vi "Configured Acquisition Trigger (Host)_20230131.vi"() -> ()   [LabVIEW 2021]
doc: "Use this VI as a template to design an application that acquires data using advanced triggering logic from the NI PXIe-5170R/5171R."
uses:
  <instrlib>/_niInstr/Multirecord Acquisition/Interface/v1/Host/Public/Full Record Status.ctl
  <instrlib>/_niInstr/Multirecord Acquisition/Interface/v1/Host/Public/Record State.ctl
  <instrlib>/_niInstr/Multirecord Acquisition/Interface/v1/Host/Public/Record Status.ctl
  Enums/Channel Numbers.ctl
  <instrlib>/_niInstr/Multirecord Acquisition/Interface/v1/Host/Public/Fetch Relative To Enum.ctl
  <vilib>/FPGAPlugInAG/PXIe-5172 (8CH - 410T)/niLvFpga_Open_PXIe-5172 (8CH - 410T).vi
  <vilib>/rvi/interface/common/dynamic/niFpgaDynamicAddResources.vi
  <vilib>/FPGAPlugInAG/Dynamic/niLvFpga_Close_Dynamic.vi
  <vilib>/rvi/interface/nirviOpenFPGA/nirviOpenFPGA.xnode
  FPGA Bitfiles/Multirecord Acquisition FPGA_20221228a_5.lvbitx
  <vilib>/rvi/interface/nirviCloseFPGA/nirviCloseFPGA.xnode
  Device Session/Device Session.lvclass
  <instrlib>/_niInstr/Multirecord Acquisition/Interface/v1/Host/niInstr Multirecord Acquisition v1 Host.lvclass
panel:
  in  "Increment Records":bool
  out "records done":u64[](array[numeric])
  out "current record status":T1
  out "fetch backlog":u64[](array[numeric])
  out "record status":T2
  out "done":bool
  out "Host Loop Count":i32
  out "Graph 1":T4(graph)
  out "TrigCfg Array":T5(array[cluster])
  out "TrigCount":u32[](array[numeric])
  in  "ResetTrig":bool=TRUE
  in  "Sliding Window Trigger":cluster{"Range":dbl, "StartCenter":dbl}[](array[cluster])=[{"Range"=0.2, "StartCenter"=0.0}, {"Range"=0.2, "StartCenter"=0.0}]
  out "actual sample rate":dbl format="%#_6p"
  in  "onboard sample clock rate":dbl(ring)=200000000.0 items=["250 MHz"=250000000.0, "200 MHz"=200000000.0, "150 MHz"=150000000.0]
  in  "impedance":enum8{"Default", "1 mega ohm", "50 ohm"}(ring)
  in  "vertical offset (V)":dbl format="%.2p"
  out "Graph 0":T4(graph)
  in  "mode":T6(ring)
  in  "decimation factor":u16=1
  in  "coupling":enum8{"Default", "DC", "AC"}(ring)
  in  "bandwidth":T7(ring)
  in  "pretrigger samples":u64=500
  in  "number of samples":u64=1000
  in  "RIO Device":tag="PXI1Slot8"
  in  "channel(s)":string="0,1"
  in  "vertical range (Vpp)":dbl=2.0 format="%.2p"
  out "error out":errorcluster
  in  "stop":bool
  # "RIO Device"
  # "Vertical Settings"
  # "Trigger Settings"
  # "Acquisition Settings"
  # "DSP"
  # "Clocking"
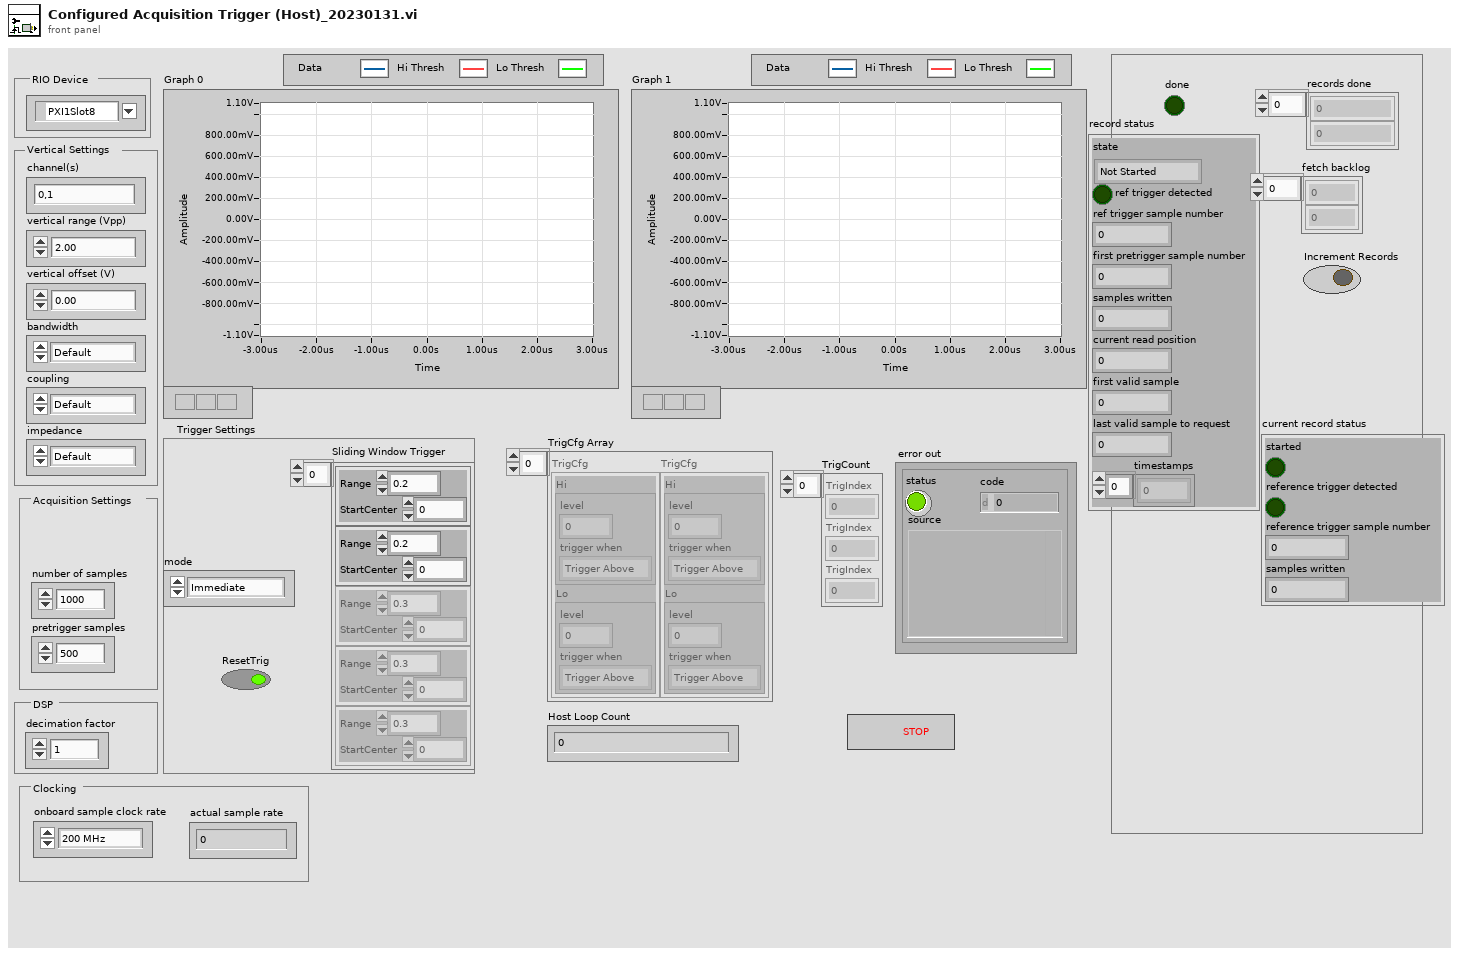
[diagram p1: front panel]
types:
  T1 = typedef "niInstr Multirecord Acquisition v1 Host.lvclass/Record Status.ctl" = cluster{"started":bool, "reference trigger detected":bool, "reference trigger sample number":u64, "samples written":u64}
  T2 = typedef "niInstr Multirecord Acquisition v1 Host.lvclass/Full Record Status.ctl" = cluster{"state":T3, "ref trigger detected":bool, "ref trigger sample number":u64, "first pretrigger sample number":u64, "samples written":u64, "current read position":u64, "first valid sample":u64, "last valid sample to request":u64, "timestamps":u64[]}
  T3 = typedef "niInstr Multirecord Acquisition v1 Host.lvclass/Record State.ctl" = enum16{"Not Started", "Being Acquired", "Completed", "Overwritten"}
  T4 = cluster{"relativeX":dbl, "sample rate":dbl, "data in":dbl[]}[]
  T5 = cluster{"Hi":cluster{"level":fxp<+/-,18,5>, "trigger when":enum8{"Trigger Above", "Trigger Below"}}, "Lo":cluster{"level":fxp<+/-,18,5>, "trigger when":enum8{"Trigger Above", "Trigger Below"}}}[]
  T6 = enum16{"Immediate", "A", "B", "OR", "AND", "A THEN B", "B THEN A", "High Resolution"}
  T7 = enum8{"Default", "Full Bandwidth", "Anti-alias Filter", "80 MHz FIR Filter", "40 MHz FIR Filter", "20 MHz FIR Filter"}
  T8 = typedef "Channel Numbers.ctl" = enum16{"0", "1", "2", "3", "4", "5", "6", "7"}
  T9 = typedef "niInstr Multirecord Acquisition v1 Host.lvclass/Fetch Relative To Enum.ctl" = enum16{"First Sample", "Reference Trigger Sample", "First Pretrigger Sample", "Most Recent Sample", "Current Read Position"}
  T10 = typedef "niInstr Multirecord Acquisition v1 Host.lvclass/Scaling Coefficient.ctl" = cluster{"gain":dbl, "offset":dbl}
  T11 = typedef "ChannelWindowClust.ctl" = cluster{"HalfRange":fxp<+/-,18,5>, "StartCenter":fxp<+/-,18,5>}
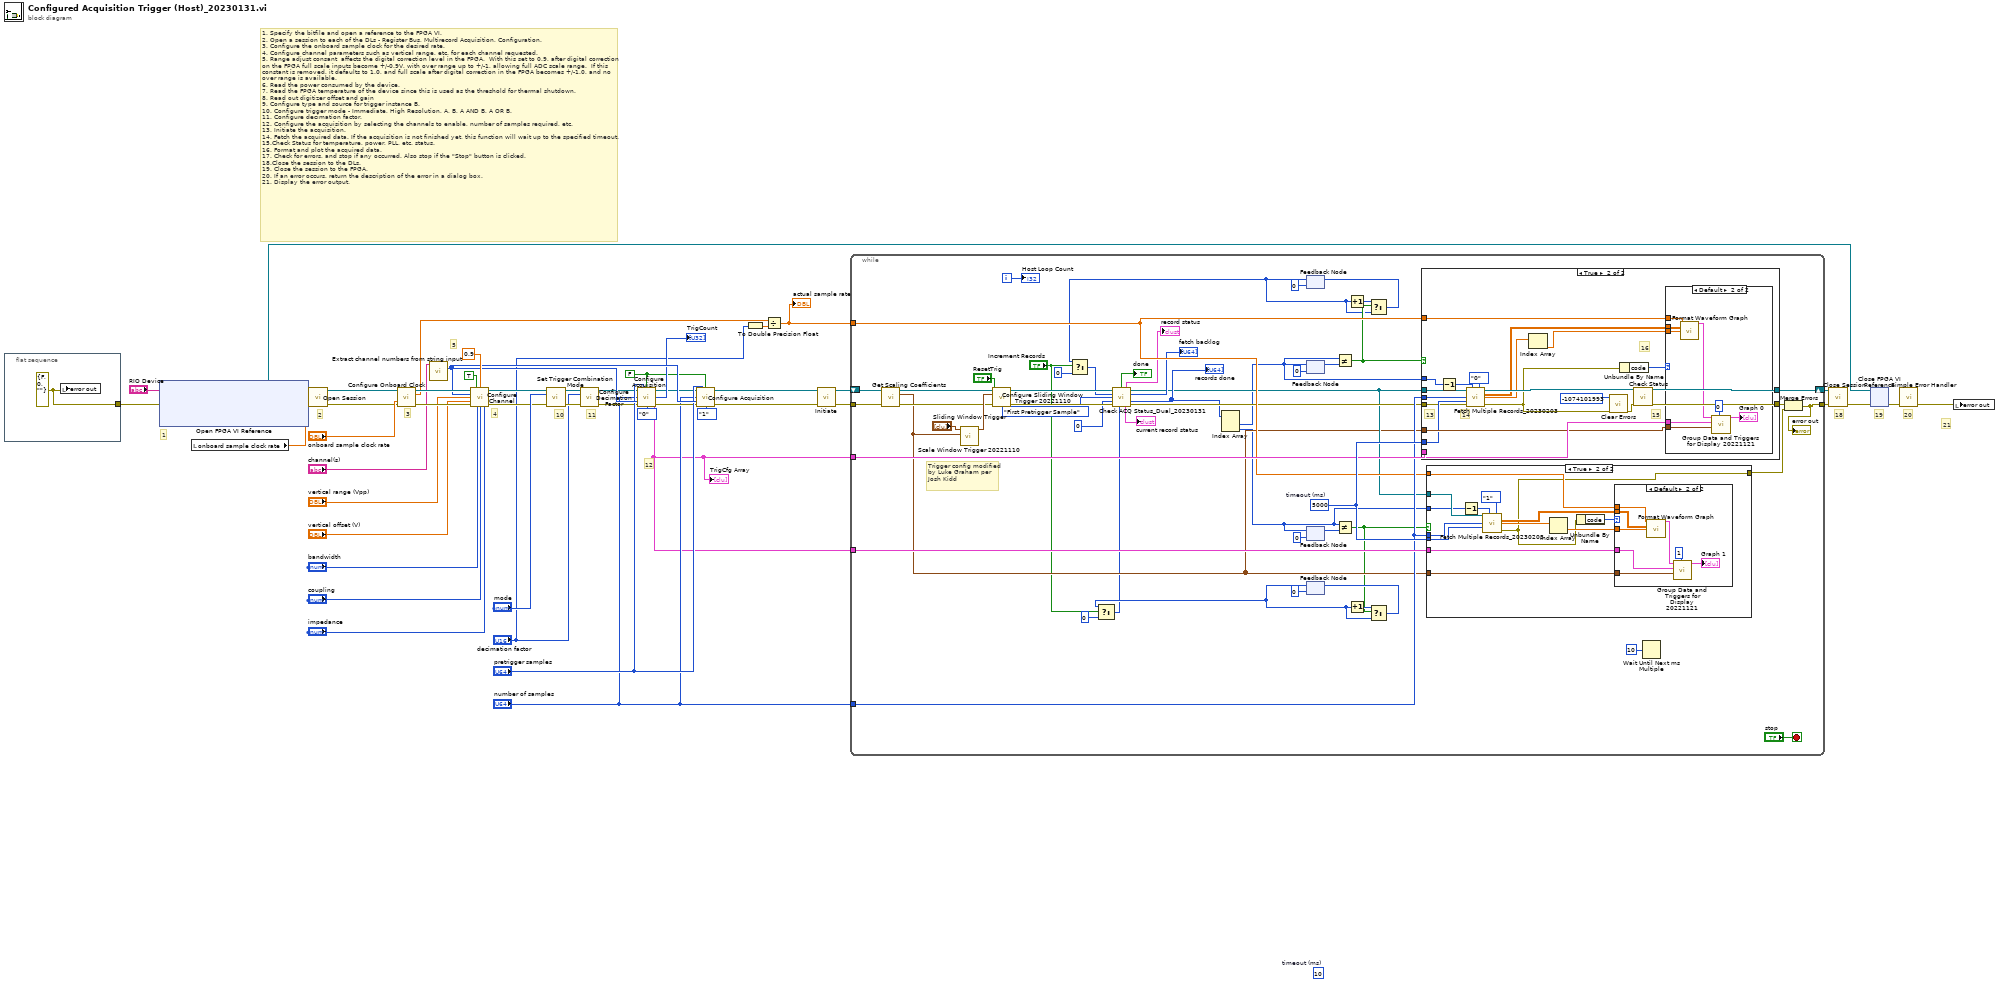
[diagram p0: block diagram]
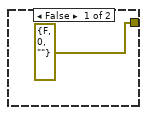
[diagram p2: hidden frame]
diagram:
  w1 = FALSE ("number of records is finite (T)")
  (unwired) 10  # timeout (ms)
  # "11"
  # "10"
  # "12"
  # "4"
  # "5"
  # "3"
  # "21"
  # "20"
  # "19"
  # "18"
  # "1. Specify the bitfile and open a reference to the FPGA VI.\n2. Open a session to each of the DLs - Register Bus, Multirecord Acquisition, Configuration.\n3. Configure the onboard sample clock for the desired rate.\n4. Configure channel parameters such as vertical range, etc. for each channel requested.\n5. Range adjust consant  affects the digital correction level in the FPGA.  With this set to 0.9, after digital correction\non the FPGA full scale inputs become +/-0.9V, with over range up to +/-1, allowing full ADC scale range.  If this \nconstant is removed, it defaults to 1.0, and full scale after digital correction in the FPGA becomes +/-1.0, and no\nover range is available.  \n6. Read the power consumed by the device.\n7. Read the FPGA temperature of the device since this is used as the threshold for thermal shutdown.\n8. Read out digitizer offset and gain\n9. Configure type and source for trigger instance B.\n10. Configure trigger mode - Immediate, High Resolution, A, B, A AND B, A OR B.\n11. Configure decimation factor.\n12. Configure the acquisition by selecting the channels to enable, number of samples required, etc.\n13. Initiate the acquisition.\n14. Fetch the acquired data. If the acquisition is not finished yet, this function will wait up to the specified timeout.\n15.Check Status for temperature, power, PLL, etc. status. \n16. Format and plot the acquired data.\n17. Check for errors, and stop if any occurred. Also stop if the \"Stop\" button is clicked.\n18.Close the session to the DLs.\n19. Close the session to the FPGA.\n20. If an error occurs, return the description of the error in a dialog box.\n21. Display the error output."
  # "2"
  # "1"
  n1 = flat-sequence {
    tunnel: [w49] -> w40
    frame #0 {
      w49 = errorcluster {"status"=FALSE, "code"=0, "source"=""} ("error constant")
      n2 = local write "error out"(w49) -> ()
    }
  }
  n3 = xnode "Open FPGA VI Reference"("error in"=w40, "resource name"="RIO Device") -> ("FPGA VI Reference Out"=w44:refnum<k20>, "error out"=w39:errorcluster)
  n4 = local read "onboard sample clock rate"() -> (w42:dbl)
  n5 = call "Open Session.vi"("FPGA Ref"=w44, "adc clock rate (Hz)"=w42, "error in"=w39) -> ("device session out"=w29:refnum<class "Device Session.lvclass">, "error out"=w28:errorcluster)  [unwired: 11 in]
  n6 = call "Configure Onboard Clock.vi"("device session in"=w29, "adc clock rate (Hz)"="onboard sample clock rate", "error in"=w28) -> ("device session out"=w38:refnum<class "Device Session.lvclass">, "actual adc clock rate (Hz)"=w6:dbl, "error out"=w33:errorcluster)  [unwired: 9 in, 1 out]
  n7 = call "Extract channel numbers from string input.vi"("channel input"="channel(s)") -> ("array of chans"=w25:u32[])  [unwired: 13 in, 1 out]
  n8 = call "Configure Channel.vi"("device session in"=w38, "enable channel (T)"=TRUE ("enable channel"), "range adjust"=0.9, "channels"=w25, "vertical range (Vpp)"="vertical range (Vpp)", "vertical offset (V)"="vertical offset (V)", "error in"=w33, "bandwidth"="bandwidth", "coupling"="coupling", "impedance"="impedance") -> ("device session out"=w13:refnum<class "Device Session.lvclass">, "error out"=w12:errorcluster)  [unwired: 4 in]
  n9 = call "Set Trigger Combination Mode.vi"("device session in"=w13, "mode"="mode", "error in"=w12) -> ("device session out"=w16:refnum<class "Device Session.lvclass">, "error out"=w17:errorcluster)  [unwired: 11 in]
  n10 = call "Configure Decimation Factor.vi"("device session in"=w16, "decimation factor"="decimation factor", "error in"=w17) -> ("device session out"=w19:refnum<class "Device Session.lvclass">, "error out"=w18:errorcluster)  [unwired: 11 in]
  n11 = call "Configure Acquisition.vi"("device session in"=w19, "pretrigger samples"="pretrigger samples", "number of records is finite (T)"=w1, "number of samples"="number of samples", "channels to store"=w25, "error in"=w18, "Chan#"=Channel_Numbers."0") -> ("device session out"=w20:refnum<class "Device Session.lvclass">, "TrigCount"=→"TrigCount":u32[], "TrigCfg Array"=w4:T5, "error out"=w21:errorcluster)  [unwired: 4 in, 1 out]
  "TrigCfg Array" <- w4
  n12 = call "Configure Acquisition.vi"("device session in"=w20, "pretrigger samples"="pretrigger samples", "number of records is finite (T)"=w1, "number of samples"="number of samples", "channels to store"=w25, "error in"=w21, "Chan#"=Channel_Numbers."1") -> ("device session out"=w3:refnum<class "Device Session.lvclass">, "error out"=w2:errorcluster)  [unwired: 4 in, 3 out]
  n13 = To Double Precision Float(number="decimation factor") -> (double precision float=w8:dbl)
  n14 = Divide(x=w6, y=w8) -> (x/y=w7:dbl)
  "actual sample rate" <- w7
  n15 = call "Initiate.vi"("device session in"=w3, "error in"=w2) -> ("device session out"=w10:refnum<class "Device Session.lvclass">, "error out"=w9:errorcluster)  [unwired: 12 in]
  n16 = while {
    shift-right: [w100] -> w47
    shift-left: w10 -> [w53]
    tunnel: [w82] -> w48
    tunnel: w9 -> [w54]
    tunnel: w4 -> [w96]
    tunnel: w4 -> [w95]
    tunnel: "number of samples" -> [w94]
    tunnel: w7 -> [w93]
    i -> [w97]
    stop <- "stop" stop-if-true
    w98 = 5000  # timeout (ms)
    # "Trigger config modified by Luke Graham per Josh Kidd"
    n17 = call "Get Scaling Coefficients.vi"("device session in"=w53, "error in"=w54) -> ("device session out"=w75:refnum<class "Device Session.lvclass">, "scaling coefficients"=w74:T10[], "error out"=w76:errorcluster)  [unwired: 11 in]
    n18 = call "Scale Window Trigger 20221110.vi"("scaling coefficients"=w74, "Sliding Window Trigger"="Sliding Window Trigger") -> ("Sliding Window Trigger (FXP)"=w77:T11[])  [unwired: 9 in]
    n19 = call "Configure Sliding Window Trigger 20221110.vi"("device session in"=w75, "Sliding Window Triggers (FXP)"=w77, "ResetTrig"="ResetTrig", "error in"=w76) -> ("device session out"=w73:refnum<class "Device Session.lvclass">, "error out"=w72:errorcluster)  [unwired: 10 in]
    n20 = feedback #1(u64 0 ("record count 0")) -> (w62:u64)
    n21 = Select(t=w62, s="Increment Records", f=u64 0) -> (s? t:f=w50:u64)
    n22 = feedback #2(u64 0 ("records done 0")) -> (w85:u64)
    n23 = feedback #3(u64 0 ("records done 0")) -> (w81:u64)
    n24 = feedback #4(u64 0 ("record count 0")) -> (w59:u64)
    n25 = Select(t=w59, s="Increment Records", f=u64 0) -> (s? t:f=w58:u64)
    n26 = call "Check ACQ Status_Dual_20230131.vi"("Device Session.lvclass"=w73, "record count 0"=w50, "fetch relative to"=Fetch_Relative_To_Enum."First Pretrigger Sample", "fetch offset"=i64 0, "error in"=w72, "record count 1"=w58) -> ("done"=→"done":bool, "record status"=→"record status":T2, "Device Session.lvclass 2"=w84:refnum<class "Device Session.lvclass">, "fetch backlog"=→"fetch backlog":u64[], "records done"=w87:u64[], "current record status"=→"current record status":T1, "error out"=w92:errorcluster)  [unwired: 1 in, 2 out]
    "records done" <- w87
    n27 = Index Array(array=w87) -> (element #1=w56:u64, element #2=w55:u64)  [unwired: 2 in]
    n28 = feedback-in #2(w56) -> ()
    n29 = feedback-in #3(w55) -> ()
    n30 = Not Equal?(x=w56, y=w85) -> (x != y?=w67:bool)
    n31 = Not Equal?(x=w55, y=w81) -> (x != y?=w52:bool)
    n32 = Increment(x=w62) -> (x+1=w68:u64)
    n33 = Increment(x=w59) -> (x+1=w64:u64)
    n34 = Select(t=w68, s=w67, f=w62) -> (s? t:f=w66:u64)
    n35 = feedback-in #1(w66) -> ()
    n36 = Select(t=w64, s=w52, f=w59) -> (s? t:f=w65:u64)
    n37 = feedback-in #4(w65) -> ()
    n38 = case shown="True" w67 {
      tunnel: [w125 w146] -> w100
      tunnel: [w126 w145] -> w99
      tunnel: w98 -> [_ w136]
      tunnel: w95 -> [_ w141]
      tunnel: w94 -> [_ w137]
      tunnel: w74 -> [_ w140]
      tunnel: w93 -> [_ w139]
      tunnel: w84 -> [w125 w130]
      tunnel: w92 -> [w126 w134]
      tunnel: w56 -> [_ w128]
      frame False {
      }
      frame True {
        # "15"
        # "16"
        # "14"
        # "13"
        n39 = Decrement(x=w128) -> (x-1=w127:u64)
        n40 = call "Fetch Multiple Records_20230203.vi"("device session in"=w130, "starting record"=w127, "Chan#"=Channel_Numbers."0", "number of samples"=w137, "timeout (ms)"=w136, "error in"=w134) -> ("device session out"=w138:refnum<class "Device Session.lvclass">, "data"=w131:dbl[][], "relativeX (samples)"=w132:dbl[], "error out"=w135:errorcluster)  [unwired: 5 in, 1 out]
        n41 = Index Array(array=w132) -> (element=w129:dbl)  [unwired: 1 in]
        n42 = call <vilib>:"Clear Errors.vi"("error in (no error)"=w135, "specific error code to clear (0: all)"=-1074101993) -> ("error out"=w143:errorcluster)  [unwired: 4 in, 1 out]
        n43 = Unbundle By Name(w135) -> ("code"=w144:i32)
        n44 = call "Check Status.vi"("device session in"=w138, "error in"=w143) -> ("device session out"=w146:refnum<class "Device Session.lvclass">, "error out"=w145:errorcluster)  [unwired: 12 in]
        n45 = case shown="Default" w144 {
          tunnel: w141 -> [_ w152]
          tunnel: w140 -> [_ w153]
          tunnel: w139 -> [_ w151]
          tunnel: w131 -> [_ w150]
          tunnel: w129 -> [_ w149]
          frame -1074101998, -1074101995, -1074101993 {
          }
          frame Default {
            n46 = call "Format Waveform Graph.vi"("sample rate (Hz)"=w151, "data in"=w150, "relativeX (samples)"=w149) -> ("waveform out"=w148:T4)  [unwired: 12 in]
            n47 = call "Group Data and Triggers for Display 20221121.vi"("Chan"=0, "scaling coefficients"=w153, "TrigCfg"=w152, "Data waveform"=w148) -> ("Data for Display"=→"Graph 0":T4)  [unwired: 7 in]
          }
        }
      }
    }
    n48 = case shown="True" w52 {
      tunnel: w98 -> [_ w110]
      tunnel: w96 -> [_ w115]
      tunnel: w94 -> [_ w111]
      tunnel: w74 -> [_ w114]
      tunnel: w93 -> [_ w113]
      tunnel: w84 -> [_ w112]
      tunnel: [errorcluster {"status"=FALSE, "code"=0, "source"=""} ("error out") w105] -> w83
      tunnel: w55 -> [_ w103]
      frame False {
      }
      frame True {
        n49 = Decrement(x=w103) -> (x-1=w104:u64)
        n50 = call "Fetch Multiple Records_20230203.vi"("device session in"=w112, "starting record"=w104, "Chan#"=Channel_Numbers."1", "number of samples"=w111, "timeout (ms)"=w110) -> ("data"=w109:dbl[][], "relativeX (samples)"=w108:dbl[], "error out"=w105:errorcluster)  [unwired: 6 in, 2 out]
        n51 = Index Array(array=w108) -> (element=w107:dbl)  [unwired: 1 in]
        n52 = Unbundle By Name(w105) -> ("code"=w116:i32)
        n53 = case shown="Default" w116 {
          tunnel: w109 -> [_ w123]
          tunnel: w115 -> [_ w124]
          tunnel: w114 -> [_ w120]
          tunnel: w107 -> [_ w118]
          tunnel: w113 -> [_ w117]
          frame -1074101998, -1074101995, -1074101993 {
          }
          frame Default {
            n54 = call "Format Waveform Graph.vi"("sample rate (Hz)"=w117, "data in"=w123, "relativeX (samples)"=w118) -> ("waveform out"=w122:T4)  [unwired: 12 in]
            n55 = call "Group Data and Triggers for Display 20221121.vi"("Chan"=1, "scaling coefficients"=w120, "TrigCfg"=w124, "Data waveform"=w122) -> ("Data for Display"=→"Graph 1":T4)  [unwired: 7 in]
          }
        }
      }
    }
    n56 = Wait Until Next ms Multiple(millisecond multiple=u32 10) -> ()  [unwired: 1 out]
    n57 = Merge Errors(w99, w83) -> (w82:errorcluster)
    "error out" <- w82
    "Host Loop Count" <- w97
  }
  n58 = call "Close Session.vi"("device session in"=w47, "error in"=w48) -> ("error out"=w45:errorcluster)  [unwired: 13 in]
  n59 = xnode "Close FPGA VI Reference"("FPGA VI Reference In"=w44, "error in"=w45) -> ("error out"=w43:errorcluster)
  n60 = call <vilib>:"Simple Error Handler.vi"("error in (no error)"=w43) -> ("error out"=w41:errorcluster)  [unwired: 4 in, 4 out]
  n61 = local write "error out"(w41) -> ()
